vi "Controle_Manip_Main_GUI_Backup2.vi"() -> ()   [LabVIEW 2019] (continued)
                            # "measurement"
                            n1619 = local read "ESP 301 On?"() -> (w2075:bool)
                            n1620 = case shown="True" w2075 {
                              frame False {
                                n1621 = local read "Log file"() -> (w2079:string)
                                n1622 = call "Write2LogFile.vi"("Add to log file"="ESP301 not activated", "Log file before"=w2079, "Checkbox"=FALSE) -> ("Log file after"=w2078:string)
                                n1623 = local write "Log file"(w2078) -> ()
                              }
                              frame True {
                                n1624 = stacked-sequence {
                                frame #0 {
                                # "get refs and exp params"
                                n1625 = local read "LightField Automation out"() -> (w2090:refnum<class "LightField Automation.lvclass">)
                                n1626 = local read "Photodiode error out"() -> (w2085:errorcluster)
                                n1627 = local read "LightField Automation error out"() -> (w2089:errorcluster)
                                n1628 = local read "ESP 301 COM Port"() -> (w2088:refnum<visa-resource-name>)
                                n1629 = local read "Photodiode handle out"() -> (w2086:refnum<visa-resource-name>)
                                n1630 = local read "ESP 301 Error"() -> (w2087:errorcluster)
                                n1631 = property on="Full scale" class="Bool (strict)"("Val(Sgnl)"=TRUE ("Value (Signaling)")) -> ()  [unwired: 2 in, 2 out]
                                n1632 = Bundle("LightField Automation out"=w2090, "LightField Automation error out"=w2089, "ESP 301 COM Port"=w2088, "ESP 301 Error"=w2087, "Photodiode handle out"=w2086, "Photodiode error out"=w2085) -> (→"Test Handles Polar":T16)  [unwired: 1 in]
                                n1633 = local read "CCD ROI"() -> (w2081:T20)
                                n1634 = local read "Exposure Time (ms)"() -> (w2092:dbl)
                                n1635 = local read "Polar Start Angle (°)"() -> (w2096:dbl)
                                n1636 = local read "Polar Step Angle (°)"() -> (w2095:dbl)
                                n1637 = local read "Polar End Angle (°)"() -> (w2091:dbl)
                                n1638 = local read "KCube Shutter On?"() -> (w2084:bool)
                                n1639 = local read "Polar mode"() -> (w2093:u16)
                                n1640 = local read "Acq Mode"() -> (w2094:T3)
                                n1641 = Bundle("Polar End Angle (°)"=w2091, "Polar Start Angle (°)"=w2096, "Polar Step Angle (°)"=w2095, "Acq Mode"=w2094, "Polar mode"=w2093, "Exposure Time (ms)"=w2092, "CCD ROI"=w2081, "KCube Shutter On?"=w2084) -> (→"Polar Params SubVIv2":T15)  [unwired: 1 in]
                                }
                                frame #1 {
                                # "Prepare graph and controls"
                                n1642 = local read "Scan Polarisation References"() -> (w2100:T17)
                                n1643 = local read "Polar Params SubVIv2"() -> (w2101:T15)
                                n1644 = local read "Scan Polar Params"() -> (w2102:refnum<vi>[])
                                n1645 = call "SubVI_PrePolarisation.vi"("Test References"=w2100, "Polar Params SubVIv2"=w2101, "Scan Polar Params"=w2102) -> ()
                                n1646 = property on="Elapsed (s)" class="DigNum (strict)"("Visible"=TRUE) -> ()  [unwired: 2 in, 2 out]
                                n1647 = property on="CCD 1D Spectrum Main" class="XYGraph (strict)"() -> ("XScale.Maximum"=w2105:dbl, "XScale.Minimum"=w2104:dbl, "YScale.Minimum"=w2099:dbl, "YScale.Maximum"=w2103:dbl)  [unwired: 2 in, 2 out]
                                n1648 = property on="Experiment Graph Controls" class="TabCtl (strict)"("Value"=T25."Polar" ("Experiment Graph Controls")) -> ()  [unwired: 2 in, 2 out]
                                n1649 = property on="Polarisation 1D Spectrum" class="XYGraph (strict)"("XScale.Maximum"=w2105, "XScale.Minimum"=w2104, "YScale.Minimum"=w2099, "YScale.Maximum"=w2103) -> ()  [unwired: 2 in, 2 out]
                                }
                                frame #2 {
                                # "actual exp"
                                n1650 = local read "Scan Polarisation References"() -> (w2112:T17)
                                n1651 = local read "Polar Params SubVIv2"() -> (w2113:T15)
                                n1652 = local read "Test Handles Polar"() -> (w2111:T16)
                                n1653 = call "Polarisation_v2.vi"("Test Handles Polar"=w2111, "Polar Params SubVIv2"=w2113, "Test References"=w2112) -> ("2D Pol Data"=w2110:dbl[][], "Test Handles Out"=w2108:T35, "Angles"=w2109:dbl[], "Wavelengths"=w2106:dbl[], "Puissances"=→"PuissancesPolar":dbl[])  [unwired: 1 in]
                                n1654 = local write "Test Handles Polar"(w2108) -> ()
                                n1655 = local write "Angles"(w2109) -> ()
                                n1656 = local write "Wavelength calibration"(w2106) -> ()
                                n1657 = local write "Pol 2D Array Out"(w2110) -> ()
                                }
                                frame #3 {
                                n1658 = control-ref of="MasterStop"() -> (w2115:refnum<vi>)
                                n1659 = control-ref of="MasterPause"() -> (w2116:refnum<vi>)
                                n1660 = control-ref of="ExperimentStopped?"() -> (w2114:refnum<vi>)
                                n1661 = call "CheckStopAndReset.vi"("ExperimentStopped?"=w2114, "MasterStop"=w2115, "MasterPause"=w2116) -> ()
                                }
                                frame #4 {
                                # "end exp"
                                n1662 = local read "Scan Polarisation References"() -> (w2122:T17)
                                n1663 = local read "Scan Polar Params"() -> (w2123:refnum<vi>[])
                                n1664 = local read "Angles"() -> (w2124:dbl[])
                                n1665 = local read "Test Handles Polar"() -> (w2121:T16)
                                n1666 = call "SubVI_PostPolarisation.vi"("Test References"=w2122, "Angles"=w2124, "Scan Polar Params"=w2123) -> ()
                                n1667 = Unbundle By Name(w2121) -> ("LightField Automation out"=w2120:refnum<class "LightField Automation.lvclass">, "LightField Automation error out"=w2119:errorcluster)
                                n1668 = property on="Elapsed (s)" class="DigNum (strict)"("Visible"=FALSE) -> ()  [unwired: 2 in, 2 out]
                                n1669 = local write "LightField Automation error out"(w2119) -> ()
                                n1670 = local write "LightField Automation out"(w2120) -> ()
                                n1671 = property on="Experiment Graph Controls" class="TabCtl (strict)"("Value"=T25."Polar" ("Experiment Graph Controls")) -> ()  [unwired: 2 in, 2 out]
                                }
                                }
                              }
                            }
                          }
                        }
                      }
                      frame "Acquire Contrast" {
                        n1672 = stacked-sequence {
                          frame #0 {
                            # "background"
                            n1673 = local read "Background taken?"() -> (w2125:bool)
                            n1674 = case shown="False" w2125 {
                              frame False {
                                n1675 = stacked-sequence {
                                tunnel: [_ _ w2175] -> w2126
                                frame #0 {
                                n1676 = local read "Log file"() -> (w2160:string)
                                n1677 = property on="CCD 1D Spectrum Main" class="XYGraph (strict)"("YScale.Offset"=0.0 ("Y Scale.Offset and Multiplier:Offset")) -> ()  [unwired: 2 in, 2 out]
                                n1678 = call "Write2LogFile.vi"("Add to log file"="Acquiring background", "Log file before"=w2160, "Checkbox"=FALSE) -> ("Log file after"=w2159:string)
                                n1679 = local write "Log file"(w2159) -> ()
                                }
                                frame #1 {
                                # "make sure shutter is closed"
                                n1680 = local read "KCube Shutter On?"() -> (w2161:bool)
                                n1681 = control-ref of="Shutter Ctrls"() -> (w2165:refnum<vi>)
                                n1682 = property class="Ring (strict)"(reference=w2165) -> ("Value"=w2164:u16)  [unwired: 1 in, 2 out]
                                n1683 = control-ref of="KCube Shutter Device Reference"() -> (w2166:refnum<vi>)
                                n1684 = Equal?(x=w2164, y=u16 0) -> (x = y?=w2162:bool)
                                n1685 = case shown="False" w2162 {
                                tunnel: w2166 -> [w2169 _]
                                tunnel: w2165 -> [w2168 _]
                                tunnel: w2161 -> [w2167 _]
                                frame False {
                                n1686 = call "Shutter.vi"("KCube Shutter Device Reference 2"=w2169, "Shutter Ctrls 2"=w2168, "Shutter on?"=w2167) -> ()
                                }
                                frame True {
                                }
                                }
                                }
                                frame #2 {
                                # "acquire"
                                n1687 = local read "LightField Automation error out"() -> (w2173:errorcluster)
                                n1688 = local read "LightField Automation out"() -> (w2174:refnum<class "LightField Automation.lvclass">)
                                n1689 = local read "Accumulations"() -> (w2170:dbl)
                                n1690 = call "LFA_Capture.vi"("error in (no error)"=w2173, "Frames"=w2170, "LightField Automation in"=w2174) -> ("error out"=w2172:errorcluster, "Data"=w2175:T26, "LightField Automation out"=w2171:refnum<class "LightField Automation.lvclass">)  [unwired: 6 in]
                                n1691 = local write "LightField Automation error out"(w2172) -> ()
                                n1692 = local write "LightField Automation out"(w2171) -> ()
                                }
                                }
                                n1693 = local read "Acq Mode"() -> (w2127:T3)
                                n1694 = case shown="\"Spectrum\", Default" w2127 {
                                selector: w2127 -> [w2128 w2146]
                                tunnel: w2126 -> [w2129 w2147]
                                frame "Spectrum", Default {
                                n1695 = stacked-sequence {
                                tunnel: w2129 -> [_ w2140 _ _]
                                tunnel: w2128 -> [_ w2138 _ _]
                                frame #0 {
                                n1696 = property on="CCD 2D Image Main" class="IntGraph (strict)"("Visible"=FALSE) -> ()  [unwired: 2 in, 2 out]
                                n1697 = property on="CCD 1D Spectrum Main" class="XYGraph (strict)"("Visible"=TRUE) -> ()  [unwired: 2 in, 2 out]
                                }
                                frame #1 {
                                n1698 = local read "Wavelength calibration"() -> (w2137:dbl[])
                                n1699 = local read "CCD ROI"() -> (w2133:T20)
                                n1700 = Divide(x=1239.842, y=w2137) -> (x/y=w2135:dbl[])
                                n1701 = call "PrepareData4Graph.vi"("Wavelength nm"=w2135, "DataLF"=w2140, "CCD ROI"=w2133, "AcqMode"=w2138, "Data type"=T30."Spectre") -> ("Spectrum"=w2139:cluster{"Array 2":dbl[], "Array":dbl[]}, "PLInt out"=w2132:dbl[])  [unwired: 2 in, 2 out]
                                n1702 = local write "CCD 1D Spectrum Main"(w2139) -> ()
                                n1703 = local write "BackgroundSpec"(w2132) -> ()
                                }
                                frame #2 {
                                n1704 = local read "BackgroundSpec"() -> (w2141:dbl[])
                                n1705 = call-poly <vilib>:"Mean.vi"("X"=w2141) -> ("mean"=w2143:dbl)  [unwired: 1 out]
                                n1706 = Negate(x=w2143) -> (-x=w2142:dbl)
                                n1707 = property on="CCD 1D Spectrum Main" class="XYGraph (strict)"("YScale.Offset"=w2142) -> ()  [unwired: 2 in, 2 out]
                                }
                                frame #3 {
                                n1708 = local write "Background taken?"(TRUE ("Background taken?")) -> ()
                                n1709 = property on="Background substract" class="Enum (strict)"("Value"=enum16{"None", "Shutter"}."None" ("Background substract")) -> ()  [unwired: 2 in, 2 out]
                                }
                                }
                                }
                                frame "Image" {
                                n1710 = stacked-sequence {
                                tunnel: w2147 -> [_ w2155]
                                tunnel: w2146 -> [_ w2153]
                                frame #0 {
                                n1711 = property on="CCD 1D Spectrum Main" class="XYGraph (strict)"("Visible"=FALSE) -> ()  [unwired: 2 in, 2 out]
                                n1712 = property on="CCD 2D Image Main" class="IntGraph (strict)"("Visible"=TRUE) -> ()  [unwired: 2 in, 2 out]
                                }
                                frame #1 {
                                n1713 = local read "Wavelength calibration"() -> (w2154:dbl[])
                                n1714 = local read "CCD ROI"() -> (w2150:T20)
                                n1715 = call "PrepareData4Graph.vi"("Wavelength nm"=w2154, "DataLF"=w2155, "CCD ROI"=w2150, "AcqMode"=w2153, "Data type"=T30."Spectre") -> ("Intensity Graph"=w2152:dbl[][])  [unwired: 2 in, 3 out]
                                n1716 = local write "CCD 2D Image Main"(w2152) -> ()
                                }
                                }
                                }
                                }
                              }
                              frame True {
                              }
                            }
                          }
                          frame #1 {
                            # "measurement"
                            n1717 = stacked-sequence {
                              frame #0 {
                                w2178 = FALSE ("Value")
                                w2179 = TRUE ("Visible")
                                w2183 = FALSE
                                w2188 = FALSE ("Acq Cont")
                                n1718 = property on="CCD 1D Spectrum Main" class="XYGraph (strict)"() -> ("XScale.Maximum"=w2187:dbl, "XScale.Minimum"=w2186:dbl, "YScale.Minimum"=w2185:dbl, "YScale.Maximum"=w2184:dbl)  [unwired: 2 in, 2 out]
                                n1719 = property on="Acquire Contrast" class="Bool (strict)"("Visible"=w2183) -> ()  [unwired: 2 in, 2 out]
                                n1720 = property on="Save Contrast" class="Bool (strict)"("Visible"=w2183) -> ()  [unwired: 2 in, 2 out]
                                n1721 = property on="Contrast 1D Spectrum" class="XYGraph (strict)"("XScale.Maximum"=w2187, "XScale.Minimum"=w2186, "YScale.Minimum"=w2185, "YScale.Maximum"=w2184) -> ()  [unwired: 2 in, 2 out]
                                n1722 = local read "Scan Contrast Ctrls"() -> (w2191:refnum<vi>[])
                                n1723 = property on="Scan Linear Stage Progess Bar" class="Slide (strict)"("Visible"=TRUE, "Value"=u8 0 ("Scan Linear Stage Progess Bar")) -> ()  [unwired: 2 in, 2 out]
                                n1724 = local write "Acquire Contrast"(w2188) -> ()
                                n1725 = local write "Save Contrast"(w2188) -> ()
                                n1726 = call "Enable&Disable_Controls.vi"("Enum"=enum16{"Enabled", "Disabled", "Disabled&Grayed"}."Disabled&Grayed", "References"=w2191) -> ()  [unwired: 1 in]
                                n1727 = property on="Scan Linear Stage Progess Bar" class="Slide (strict)"("Visible"=TRUE) -> ()  [unwired: 2 in, 2 out]
                                n1728 = property on="Elapsed (s)" class="DigNum (strict)"("Visible"=TRUE) -> ()  [unwired: 2 in, 2 out]
                                n1729 = control-ref of="MasterStop"() -> (w2181:refnum<vi>)
                                n1730 = control-ref of="MasterPause"() -> (w2180:refnum<vi>)
                                n1731 = property on="Experiment Graph Controls" class="TabCtl (strict)"("Value"=T25."Contrast" ("Experiment Graph Controls")) -> ()  [unwired: 2 in, 2 out]
                                n1732 = property class="Bool (strict)"(reference=w2180, "Visible"=w2179, "Value"=w2178) -> ()  [unwired: 1 in, 2 out]
                                n1733 = property class="Bool (strict)"(reference=w2181, "Visible"=w2179, "Value"=w2178) -> ()  [unwired: 1 in, 2 out]
                              }
                              frame #1 {
                                n1734 = local read "Excitation Wavelength (nm)"() -> (w2197:dbl)
                                n1735 = local read "LinTFines Step Pos (usteps)"() -> (w2202:dbl)
                                n1736 = local read "LinTFine Start Pos (usteps)"() -> (w2203:dbl)
                                n1737 = local read "LinTFine End Pos (usteps)"() -> (w2201:dbl)
                                n1738 = local read "Exposure Time (ms)"() -> (w2199:dbl)
                                n1739 = local read "LinT Start Pos (mm)"() -> (w2206:dbl)
                                n1740 = local read "LinT Step Pos (mm)"() -> (w2205:dbl)
                                n1741 = local read "LinT End pos (mm)"() -> (w2204:dbl)
                                n1742 = local read "KCube Shutter On?"() -> (w2194:bool)
                                n1743 = local read "Accumulations"() -> (w2198:dbl)
                                n1744 = local read "Acq Mode"() -> (w2196:T3)
                                n1745 = local read "CCD ROI"() -> (w2195:T20)
                                n1746 = Bundle("LinT Start Pos (mm)"=w2206, "LinT Step Pos (mm)"=w2205, "LinT End pos (mm)"=w2204, "LinTFine Start Pos (usteps)"=w2203, "LinTFines Step Pos (usteps)"=w2202, "LinTFine End Pos (usteps)"=w2201) -> (w2200:T27)  [unwired: 1 in]
                                n1747 = Bundle("Exposure Time (ms)"=w2199, "Accumulations"=w2198, "Excitation Wavelength (nm)"=w2197, "Acq Mode"=w2196, "CCD ROI"=w2195, "KCube Shutter On?"=w2194) -> (w2193:T24)  [unwired: 1 in]
                                n1748 = local write "Scan Translation Params"(w2200) -> ()
                                n1749 = local write "Scan Translation Exp Params"(w2193) -> ()
                              }
                              frame #2 {
                                n1750 = local read "Scan Translation Exp Params"() -> (w2214:T24)
                                n1751 = local read "Scan Translation Params"() -> (w2231:T27)
                                n1752 = control-ref of="Scan Linear Stage Progess Bar"() -> ()  [unwired: 1 out]
                                n1753 = control-ref of="Stop Contrast"() -> ()  [unwired: 1 out]
                                n1754 = local read "ESP 301 COM Port"() -> (w2224:refnum<visa-resource-name>)
                                n1755 = control-ref of="Pause Contrast"() -> ()  [unwired: 1 out]
                                n1756 = control-ref of="Scan Main Progess Bar"() -> (w2213:refnum<vi>)
                                n1757 = local read "LightField Automation error out"() -> (w2211:errorcluster)
                                n1758 = local read "ESP 301 Error"() -> (w2226:errorcluster)
                                n1759 = local read "LightField Automation out"() -> (w2212:refnum<class "LightField Automation.lvclass">)
                                n1760 = control-ref of="Shutter Ctrls"() -> (w2216:refnum<vi>)
                                n1761 = control-ref of="KCube Shutter Device Reference"() -> (w2217:refnum<vi>)
                                n1762 = control-ref of="PZC Position Readout (usteps)"() -> (w2215:refnum<vi>)
                                n1763 = control-ref of="Contrast 1D Spectrum"() -> (w2218:refnum<vi>)
                                n1764 = control-ref of="Contrast Oscillations"() -> (w2219:refnum<vi>)
                                n1765 = Open VI Reference(type specifier VI Refnum (for type only)=refnum<vi> refnum ("application reference (local)"), vi path=path "C:/Users/manip/Documents/Controle_Manip_2020/subVIs/Scans/FineContrast_cleaned inputs.vi", options=256) -> (vi reference=w2229:refnum<vi>, error out=w2238:errorcluster)  [unwired: 3 in]
                                n1766 = local read "PZC200 Instrument Channel"() -> (w2230:string)
                                n1767 = call-by-ref "Wait On Asynchronous Call"(reference=w2229, error in=w2238) -> (reference out=w2237:refnum<vi>, error out=w2236:errorcluster, "PZAPos & InstPow"=w2227:dbl[][], "Spectra vs PZA"=w2234:i32[][], "LFA out"=w2210:refnum<class "LightField Automation.lvclass">, "PZC out"=w2228:string, "Photodiode out"=w2220:refnum<visa-resource-name>, "ESP 301 COM out"=w2223:refnum<visa-resource-name>, "LFA error out"=w2209:errorcluster, "PZC error out"=w2221:errorcluster, "Photodiode error out"=w2222:errorcluster, "ESP 301 error out"=w2225:errorcluster)  [unwired: 18 in]
                                n1768 = local write "PZAPos&Pow"(w2227) -> ()
                                n1769 = local write "Photodiode error out"(w2222) -> ()
                                n1770 = local write "PZC200 Instrument Channel"(w2228) -> ()
                                n1771 = local write "Contrast Array Out"(w2234) -> ()
                                n1772 = local read "PZC Error"() -> (w2235:errorcluster)
                                n1773 = local write "ESP 301 COM Port"(w2223) -> ()
                                n1774 = Close Reference(reference=w2237, error in (no error)=w2236) -> ()  [unwired: 1 out]
                                n1775 = local write "Photodiode handle out"(w2220) -> ()
                                n1776 = local read "Photodiode handle out"() -> (w2232:refnum<visa-resource-name>)
                                n1777 = local write "ESP 301 Error"(w2225) -> ()
                                n1778 = local read "Photodiode error out"() -> (w2233:errorcluster)
                                n1779 = local write "LightField Automation error out"(w2209) -> ()
                                n1780 = local write "LightField Automation out"(w2210) -> ()
                                n1781 = local write "PZC Error"(w2221) -> ()
                                n1782 = control-ref of="MasterStop"() -> (w2207:refnum<vi>)
                                n1783 = control-ref of="MasterPause"() -> (w2208:refnum<vi>)
                                n1784 = call-by-ref "Start Asynchronous Call"(reference=w2229, error in=w2238, "LFA in"=w2212, "PZC in"=w2230, "Photodiode in"=w2232, "ESP 301 COM"=w2224, "LFA error in"=w2211, "PZC error in"=w2235, "Photodiode error in"=w2233, "ESP 301 error in"=w2226, "Scan Translation Exp Params"=w2214, "PZC Pos (usteps)"=w2215, "Scan Translation Params"=w2231, "Pause button"=w2208, "Contrast Oscillations"=w2219, "Stop button"=w2207, "Contrast 1D Spectrum"=w2218, "Progess Bar"=w2213, "Shutter Device"=w2217, "Shutter"=w2216) -> ()  [unwired: 12 out]
                              }
                              frame #3 {
                                w2254 = FALSE ("Acq Cont")
                                w2251 = FALSE ("Acq Cont")
                                n1785 = local read "Auto< ?"() -> (w2249:bool)
                                n1786 = property on="Scan Linear Stage Progess Bar" class="Slide (strict)"("Visible"=FALSE, "Value"=u8 0 ("Scan Linear Stage Progess Bar")) -> ()  [unwired: 2 in, 2 out]
                                n1787 = Not(x=w2249) -> (.not. x?=w2248:bool)
                                n1788 = local write "Pause Michelson"(w2254) -> ()
                                n1789 = local write "Stop Michelson"(w2254) -> ()
                                n1790 = property on="Save Contrast" class="Bool (strict)"("Visible"=w2248) -> ()  [unwired: 2 in, 2 out]
                                n1791 = property on="Acquire Contrast" class="Bool (strict)"("Visible"=TRUE) -> ()  [unwired: 2 in, 2 out]
                                n1792 = local write "Acquire Michelson"(w2251) -> ()
                                n1793 = local write "Acquire Contrast"(w2251) -> ()
                                n1794 = local write "Save Michelson"(w2251) -> ()
                                n1795 = local read "Scan Contrast Ctrls"() -> (w2247:refnum<vi>[])
                                n1796 = property on="Elapsed (s)" class="DigNum (strict)"("Visible"=FALSE) -> ()  [unwired: 2 in, 2 out]
                                n1797 = control-ref of="MasterStop"() -> (w2244:refnum<vi>)
                                n1798 = control-ref of="MasterPause"() -> (w2245:refnum<vi>)
                                n1799 = call "Enable&Disable_Controls.vi"("Enum"=enum16{"Enabled", "Disabled", "Disabled&Grayed"}."Enabled", "References"=w2247) -> ()  [unwired: 1 in]
                                n1800 = control-ref of="ExperimentStopped?"() -> (w2243:refnum<vi>)
                                n1801 = call "CheckStopAndReset.vi"("ExperimentStopped?"=w2243, "MasterStop"=w2244, "MasterPause"=w2245) -> ()
                              }
                            }
                          }
                        }
                      }
                      frame "Acquire Michelson" {
                        n1802 = stacked-sequence {
                          frame #0 {
                            # "background"
                            n1803 = local read "Background taken?"() -> (w2255:bool)
                            n1804 = case shown="False" w2255 {
                              frame False {
                                n1805 = stacked-sequence {
                                tunnel: [_ _ w2305] -> w2256
                                frame #0 {
                                n1806 = local read "Log file"() -> (w2290:string)
                                n1807 = property on="CCD 1D Spectrum Main" class="XYGraph (strict)"("YScale.Offset"=0.0 ("Y Scale.Offset and Multiplier:Offset")) -> ()  [unwired: 2 in, 2 out]
                                n1808 = call "Write2LogFile.vi"("Add to log file"="Acquiring background", "Log file before"=w2290, "Checkbox"=FALSE) -> ("Log file after"=w2289:string)
                                n1809 = local write "Log file"(w2289) -> ()
                                }
                                frame #1 {
                                # "make sure shutter is closed"
                                n1810 = local read "KCube Shutter On?"() -> (w2291:bool)
                                n1811 = control-ref of="Shutter Ctrls"() -> (w2295:refnum<vi>)
                                n1812 = property class="Ring (strict)"(reference=w2295) -> ("Value"=w2294:u16)  [unwired: 1 in, 2 out]
                                n1813 = control-ref of="KCube Shutter Device Reference"() -> (w2296:refnum<vi>)
                                n1814 = Equal?(x=w2294, y=u16 0) -> (x = y?=w2292:bool)
                                n1815 = case shown="False" w2292 {
                                tunnel: w2296 -> [w2299 _]
                                tunnel: w2295 -> [w2298 _]
                                tunnel: w2291 -> [w2297 _]
                                frame False {
                                n1816 = call "Shutter.vi"("KCube Shutter Device Reference 2"=w2299, "Shutter Ctrls 2"=w2298, "Shutter on?"=w2297) -> ()
                                }
                                frame True {
                                }
                                }
                                }
                                frame #2 {
                                # "acquire"
                                n1817 = local read "LightField Automation error out"() -> (w2303:errorcluster)
                                n1818 = local read "LightField Automation out"() -> (w2304:refnum<class "LightField Automation.lvclass">)
                                n1819 = local read "Accumulations"() -> (w2300:dbl)
                                n1820 = call "LFA_Capture.vi"("error in (no error)"=w2303, "Frames"=w2300, "LightField Automation in"=w2304) -> ("error out"=w2302:errorcluster, "Data"=w2305:T26, "LightField Automation out"=w2301:refnum<class "LightField Automation.lvclass">)  [unwired: 6 in]
                                n1821 = local write "LightField Automation error out"(w2302) -> ()
                                n1822 = local write "LightField Automation out"(w2301) -> ()
                                }
                                }
                                n1823 = local read "Acq Mode"() -> (w2257:T3)
                                n1824 = case shown="\"Spectrum\", Default" w2257 {
                                selector: w2257 -> [w2258 w2276]
                                tunnel: w2256 -> [w2259 w2277]
                                frame "Spectrum", Default {
                                n1825 = stacked-sequence {
                                tunnel: w2259 -> [_ w2270 _ _]
                                tunnel: w2258 -> [_ w2268 _ _]
                                frame #0 {
                                n1826 = property on="CCD 2D Image Main" class="IntGraph (strict)"("Visible"=FALSE) -> ()  [unwired: 2 in, 2 out]
                                n1827 = property on="CCD 1D Spectrum Main" class="XYGraph (strict)"("Visible"=TRUE) -> ()  [unwired: 2 in, 2 out]
                                }
                                frame #1 {
                                n1828 = local read "Wavelength calibration"() -> (w2267:dbl[])
                                n1829 = local read "CCD ROI"() -> (w2263:T20)
                                n1830 = Divide(x=1239.842, y=w2267) -> (x/y=w2265:dbl[])
                                n1831 = call "PrepareData4Graph.vi"("Wavelength nm"=w2265, "DataLF"=w2270, "CCD ROI"=w2263, "AcqMode"=w2268, "Data type"=T30."Spectre") -> ("Spectrum"=w2269:cluster{"Array 2":dbl[], "Array":dbl[]}, "PLInt out"=w2262:dbl[])  [unwired: 2 in, 2 out]
                                n1832 = local write "CCD 1D Spectrum Main"(w2269) -> ()
                                n1833 = local write "BackgroundSpec"(w2262) -> ()
                                }
                                frame #2 {
                                n1834 = local read "BackgroundSpec"() -> (w2271:dbl[])
                                n1835 = call-poly <vilib>:"Mean.vi"("X"=w2271) -> ("mean"=w2273:dbl)  [unwired: 1 out]
                                n1836 = Negate(x=w2273) -> (-x=w2272:dbl)
                                n1837 = property on="CCD 1D Spectrum Main" class="XYGraph (strict)"("YScale.Offset"=w2272) -> ()  [unwired: 2 in, 2 out]
                                }
                                frame #3 {
                                n1838 = local write "Background taken?"(TRUE ("Background taken?")) -> ()
                                n1839 = property on="Background substract" class="Enum (strict)"("Value"=enum16{"None", "Shutter"}."None" ("Background substract")) -> ()  [unwired: 2 in, 2 out]
                                }
                                }
                                }
                                frame "Image" {
                                n1840 = stacked-sequence {
                                tunnel: w2277 -> [_ w2285]
                                tunnel: w2276 -> [_ w2283]
                                frame #0 {
                                n1841 = property on="CCD 1D Spectrum Main" class="XYGraph (strict)"("Visible"=FALSE) -> ()  [unwired: 2 in, 2 out]
                                n1842 = property on="CCD 2D Image Main" class="IntGraph (strict)"("Visible"=TRUE) -> ()  [unwired: 2 in, 2 out]
                                }
                                frame #1 {
                                n1843 = local read "Wavelength calibration"() -> (w2284:dbl[])
                                n1844 = local read "CCD ROI"() -> (w2280:T20)
                                n1845 = call "PrepareData4Graph.vi"("Wavelength nm"=w2284, "DataLF"=w2285, "CCD ROI"=w2280, "AcqMode"=w2283, "Data type"=T30."Spectre") -> ("Intensity Graph"=w2282:dbl[][])  [unwired: 2 in, 3 out]
                                n1846 = local write "CCD 2D Image Main"(w2282) -> ()
                                }
                                }
                                }
                                }
                              }
                              frame True {
                              }
                            }
                          }
                          frame #1 {
                            # "measurement"
                            n1847 = Get Date/Time In Seconds() -> (seconds since 1Jan1904=w2306:timestamp)
                            n1848 = stacked-sequence {
                              tunnel: w2306 -> [_ _ w2340 w2464]
                              frame #0 {
                                w2312 = TRUE
                                w2313 = FALSE ("Acq Cont")
                                w2310 = TRUE
                                w2309 = FALSE
                                w2311 = FALSE
                                # "check that range is within translation stage travel"
                                # "get params and check feasability"
                                n1849 = property on="Save Michelson" class="Bool (strict)"("Visible"=w2311) -> ()  [unwired: 2 in, 2 out]
                                n1850 = property on="Pause Michelson" class="Bool (strict)"("Visible"=w2310) -> ()  [unwired: 2 in, 2 out]
                                n1851 = property on="Save Contrast" class="Bool (strict)"("Visible"=w2311) -> ()  [unwired: 2 in, 2 out]
                                n1852 = property on="Pause Contrast" class="Bool (strict)"("Visible"=w2310) -> ()  [unwired: 2 in, 2 out]
                                n1853 = property on="Stop Contrast" class="Bool (strict)"("Visible"=w2310) -> ()  [unwired: 2 in, 2 out]
                                n1854 = property on="Acquire Michelson" class="Bool (strict)"("Visible"=w2311) -> ()  [unwired: 2 in, 2 out]
                                n1855 = property on="Stop Michelson" class="Bool (strict)"("Visible"=w2310) -> ()  [unwired: 2 in, 2 out]
                                n1856 = property on="Acquire Contrast" class="Bool (strict)"("Visible"=w2311) -> ()  [unwired: 2 in, 2 out]
                                n1857 = property on="Scan Linear Stage Progess Bar" class="Slide (strict)"("Visible"=TRUE, "Value"=u8 0 ("Scan Linear Stage Progess Bar")) -> ()  [unwired: 2 in, 2 out]
                                n1858 = property on="Scan Michelson Progess Bar" class="Slide (strict)"("Value"=u8 0 ("Scan Michelson Progess Bar"), "Visible"=TRUE) -> ()  [unwired: 2 in, 2 out]
                                n1859 = local read "Scan Contrast Ctrls"() -> (w2319:refnum<vi>[])
                                n1860 = local write "Acquire Contrast"(w2313) -> ()
                                n1861 = local write "Save Contrast"(w2313) -> ()
                                n1862 = call "Enable&Disable_Controls.vi"("Enum"=enum16{"Enabled", "Disabled", "Disabled&Grayed"}."Disabled&Grayed", "References"=w2319) -> ()  [unwired: 1 in]
                                n1863 = property on="Michelson Expected (s)" class="DigNum (strict)"("Visible"=w2312) -> ()  [unwired: 2 in, 2 out]
                                n1864 = property on="Elapsed (s)" class="DigNum (strict)"("Visible"=TRUE) -> ()  [unwired: 2 in, 2 out]
                                n1865 = property on="Experiment Graph Controls" class="TabCtl (strict)"("Value"=T25."Contrast" ("Experiment Graph Controls")) -> ()  [unwired: 2 in, 2 out]
                                n1866 = property on="Michelson Elapsed (s)" class="DigNum (strict)"("Visible"=w2312) -> ()  [unwired: 2 in, 2 out]
                                n1867 = local write "Acquire Michelson"(w2309) -> ()
                                n1868 = local write "Save Michelson"(w2309) -> ()
                              }
                              frame #1 {
                                # "check that range is within translation stage travel"
                                # "get params"
                                n1869 = local read "Excitation Wavelength (nm)"() -> (w2324:dbl)
                                n1870 = local read "Exposure Time (ms)"() -> (w2326:dbl)
                                n1871 = local read "KCube Shutter On?"() -> (w2321:bool)
                                n1872 = local read "Accumulations"() -> (w2325:dbl)
                                n1873 = local read "Acq Mode"() -> (w2323:T3)
                                n1874 = local read "CCD ROI"() -> (w2322:T20)
                                n1875 = local read "LinTFines Step Pos (usteps)"() -> (w2329:dbl)
                                n1876 = local read "LinTFine Start Pos (usteps)"() -> (w2330:dbl)
                                n1877 = local read "LinTFine End Pos (usteps)"() -> (w2328:dbl)
                                n1878 = local read "LinT Start Pos (mm)"() -> (w2333:dbl)
                                n1879 = local read "LinT Step Pos (mm)"() -> (w2332:dbl)
                                n1880 = local read "LinT End pos (mm)"() -> (w2331:dbl)
                                n1881 = Bundle("Exposure Time (ms)"=w2326, "Accumulations"=w2325, "Excitation Wavelength (nm)"=w2324, "Acq Mode"=w2323, "CCD ROI"=w2322, "KCube Shutter On?"=w2321) -> (w2320:T24)  [unwired: 1 in]
                                n1882 = Bundle("LinT Start Pos (mm)"=w2333, "LinT Step Pos (mm)"=w2332, "LinT End pos (mm)"=w2331, "LinTFine Start Pos (usteps)"=w2330, "LinTFines Step Pos (usteps)"=w2329, "LinTFine End Pos (usteps)"=w2328) -> (w2327:T27)  [unwired: 1 in]
                                n1883 = local write "Scan Translation Exp Params"(w2320) -> ()
                                n1884 = local write "Scan Translation Params"(w2327) -> ()
                              }
                              frame #2 {
                                # "pzc & inst pow"
                                # "esp pos"
                                # "data"
                                # "move ESP"
                                n1885 = local read "LightField Automation out"() -> (w2337:refnum<class "LightField Automation.lvclass">)
                                n1886 = local read "ESP 301 COM Port"() -> (w2339:refnum<visa-resource-name>)
                                n1887 = local read "LinT Start Pos (mm)"() -> (w2350:dbl)
                                n1888 = local read "ESP 301 Error"() -> (w2346:errorcluster)
                                n1889 = local read "LinT Step Pos (mm)"() -> (w2351:dbl)
                                n1890 = local read "LinT End pos (mm)"() -> (w2355:dbl)
                                n1891 = local read "LinT Start Pos (mm)"() -> (w2356:dbl)
                                n1892 = local read "LinT Step Pos (mm)"() -> (w2353:dbl)
                                n1893 = local read "LightField Automation error out"() -> (w2336:errorcluster)
                                n1894 = Subtract(x=w2355, y=w2356) -> (x-y=w2354:dbl)
                                n1895 = Divide(x=w2354, y=w2353) -> (x/y=w2352:dbl)
                                n1896 = Increment(x=w2352) -> (x+1=w2349:dbl)
                                n1897 = for {
                                N: w2349 -> [w2362]
                                tunnel: w2351 -> [w2379]
                                tunnel: w2350 -> [w2378]
                                shift-right: [w2374] -> w2347
                                shift-left: dbl[] [] -> [w2375]
                                shift-right: [w2372] -> w2335
                                shift-left: w2337 -> [w2373]
                                shift-right: [w2370] -> w2334
                                shift-left: w2336 -> [w2371]
                                shift-right: [w2368] -> w2345
                                shift-left: w2346 -> [w2369]
                                shift-right: [w2366] -> w2343
                                shift-left: dbl[][][] [] -> [w2367]
                                shift-right: [w2364] -> w2341
                                shift-left: dbl[][][] [] -> [w2365]
                                tunnel: w2340 -> [w2360]
                                shift-right: [w2357] -> w2338
                                shift-left: w2339 -> [w2358]
                                i -> [w2361]
                                stop <- w2359 stop-if-true
                                # "ESP"
                                n1898 = Multiply(x=w2361, y=w2379) -> (x*y=w2377:dbl)
                                n1899 = Add(x=w2378, y=w2377) -> (x+y=w2376:dbl)
                                n1900 = Divide(x=w2361, y=w2362) -> (x/y=w2363:dbl)
                                n1901 = stacked-sequence {
                                tunnel: w2376 -> [w2384 w2390 _ _]
                                tunnel: w2375 -> [w2386 _ _ _]
                                tunnel: [w2385 _ _ _] -> w2374
                                tunnel: w2373 -> [_ _ w2433 _]
                                tunnel: [_ _ w2432 _] -> w2372
                                tunnel: w2371 -> [_ _ w2431 _]
                                tunnel: [_ _ w2430 _] -> w2370
                                tunnel: w2369 -> [w2383 _ _ _]
                                tunnel: [w2382 _ _ _] -> w2368
                                tunnel: w2367 -> [_ _ w2402 _]
                                tunnel: [_ _ w2400 _] -> w2366
                                tunnel: w2365 -> [_ _ w2399 _]
                                tunnel: [_ _ w2397 _] -> w2364
                                tunnel: w2363 -> [_ _ _ w2443]
                                tunnel: w2362 -> [_ _ _ w2442]
                                tunnel: w2361 -> [_ _ _ w2440]
                                tunnel: w2360 -> [_ _ _ w2441]
                                tunnel: [_ _ _ w2438] -> w2359
                                tunnel: w2358 -> [w2381 _ _ _]
                                tunnel: [w2380 _ _ _] -> w2357
                                frame #0 {
                                # "pos readout"
                                n1902 = control-ref of="Newport Linear Translation Stage Position Readout (mm)"() -> (w2387:refnum<vi>)
                                n1903 = call "ESP301_Go2Pos.vi"("VISA resource name"=w2381, "Set value"=w2384, "Axis (1)"=1, "Error In"=w2383, "DigNum Refnum"=w2387) -> ("VISA resource name 2"=w2380:refnum<visa-resource-name>, "Error In 2"=w2382:errorcluster)
                                n1904 = Insert Into Array(array=w2386, new element=w2384) -> (w2385:dbl[])  [unwired: 1 in]
                                }
                                frame #1 {
                                # "wait on ESP"
                                n1905 = Wait (ms)(milliseconds to wait=u32 50) -> ()  [unwired: 1 out]
                                n1906 = Number To Decimal String(number=w2390) -> (decimal integer string=w2393:string)  [unwired: 1 in]
                                n1907 = local read "Log file"() -> (w2396:string)
                                n1908 = Concatenate Strings("ESP moved to ", w2393) -> (w2392:string)
                                n1909 = call "Write2LogFile.vi"("Add to log file"=w2392, "Log file before"=w2396, "Checkbox"=FALSE) -> ("Log file after"=w2395:string)
                                n1910 = local write "Log file"(w2395) -> ()
                                }
                                frame #2 {
                                n1911 = control-ref of="Shutter Ctrls"() -> (w2420:refnum<vi>)
                                n1912 = control-ref of="Scan Linear Stage Progess Bar"() -> (w2416:refnum<vi>)
                                n1913 = control-ref of="KCube Shutter Device Reference"() -> (w2421:refnum<vi>)
                                n1914 = control-ref of="PZC Position Readout (usteps)"() -> (w2419:refnum<vi>)
                                n1915 = control-ref of="Pause Contrast"() -> (w2418:refnum<vi>)
                                n1916 = control-ref of="Contrast 1D Spectrum"() -> (w2422:refnum<vi>)
                                n1917 = control-ref of="Contrast Oscillations"() -> (w2423:refnum<vi>)
                                n1918 = local read "Photodiode handle out"() -> (w2412:refnum<visa-resource-name>)
                                n1919 = local read "Photodiode error out"() -> (w2413:errorcluster)
                                n1920 = control-ref of="Stop Contrast"() -> (w2417:refnum<vi>)
                                n1921 = local read "Scan Translation Params"() -> (w2425:T27)
                                n1922 = Open VI Reference(type specifier VI Refnum (for type only)=refnum<vi> refnum ("application reference (local)"), vi path=path "C:/Users/manip/Documents/Controle_Manip_2020/subVIs/Scans/FineContrast_cleaned inputs.vi", options=256) -> (vi reference=w2427:refnum<vi>, error out=w2426:errorcluster)  [unwired: 3 in]
                                n1923 = local read "Scan Translation Exp Params"() -> (w2424:T24)
                                n1924 = local read "PZC200 Instrument Channel"() -> (w2411:string)
                                n1925 = local read "ESP 301 Error"() -> (w2414:errorcluster)
                                n1926 = local read "PZC Error"() -> (w2410:errorcluster)
                                n1927 = local read "ESP 301 COM Port"() -> (w2415:refnum<visa-resource-name>)
                                n1928 = call-by-ref "Start Asynchronous Call"(reference=w2427, error in=w2426, "LFA in"=w2433, "PZC in"=w2411, "Photodiode in"=w2412, "ESP 301 COM"=w2415, "LFA error in"=w2431, "PZC error in"=w2410, "Photodiode error in"=w2413, "ESP 301 error in"=w2414, "Scan Translation Exp Params"=w2424, "PZC Pos (usteps)"=w2419, "Scan Translation Params"=w2425, "Pause button"=w2418, "Contrast Oscillations"=w2423, "Stop button"=w2417, "Contrast 1D Spectrum"=w2422, "Progess Bar"=w2416, "Shutter Device"=w2421, "Shutter"=w2420) -> ()  [unwired: 12 out]
                                n1929 = call-by-ref "Wait On Asynchronous Call"(reference=w2427, error in=w2426) -> ("PZAPos & InstPow"=w2398:dbl[][], "Spectra vs PZA"=w2401:i32[][], "LFA out"=w2432:refnum<class "LightField Automation.lvclass">, "PZC out"=w2407:string, "Photodiode out"=w2406:refnum<visa-resource-name>, "ESP 301 COM out"=w2408:refnum<visa-resource-name>, "LFA error out"=w2430:errorcluster, "PZC error out"=w2404:errorcluster, "Photodiode error out"=w2405:errorcluster, "ESP 301 error out"=w2409:errorcluster)  [unwired: 18 in, 2 out]
                                n1930 = local write "PZC200 Instrument Channel"(w2407) -> ()
                                n1931 = local write "Photodiode handle out"(w2406) -> ()
                                n1932 = local write "Photodiode error out"(w2405) -> ()
                                n1933 = local write "ESP 301 COM Port"(w2408) -> ()
                                n1934 = Insert Into Array(array=w2399, new element=w2398) -> (w2397:dbl[][][])  [unwired: 3 in]
                                n1935 = local write "ESP 301 Error"(w2409) -> ()
                                n1936 = local write "PZC Error"(w2404) -> ()
                                n1937 = Insert Into Array(array=w2402, new element=w2401) -> (w2400:dbl[][][])  [unwired: 3 in]
                                }
                                frame #3 {
                                n1938 = local read "Pause Michelson"() -> (w2437:bool)
                                n1939 = control-ref of="Expected (s)"() -> (w2435:refnum<vi>)
                                n1940 = Increment(x=w2440) -> (x+1=w2439:i32)
                                n1941 = Multiply(x=w2443, y=100.0) -> (x*y=w2445:dbl)
                                n1942 = call "Expectedtime.vi"("N"=w2442, "I"=w2439, "Reference time"=w2441) -> ("Expected time"=w2434:dbl, "Elapsed time"=w2436:dbl)
                                "Michelson Elapsed (s)" <- w2436
                                "Michelson Expected (s)" <- w2434
                                n1943 = property class="DigNum (strict)"(reference=w2435, "Value"=w2434) -> ()  [unwired: 1 in, 2 out]
                                n1944 = property on="Elapsed (s)" class="DigNum (strict)"("Value"=w2436) -> ()  [unwired: 2 in, 2 out]
                                n1945 = local write "Scan Michelson Progess Bar"(w2445) -> ()
                                n1946 = case shown="True" w2437 {
                                frame False {
                                }
                                frame True {
                                n1947 = while {
                                stop <- w2447 stop-if-true
                                n1948 = local read "Pause Michelson"() -> (w2448:bool)
                                n1949 = Wait (ms)(milliseconds to wait=u32 50) -> ()  [unwired: 1 out]
                                n1950 = Not(x=w2448) -> (.not. x?=w2447:bool)
                                }
                                }
                                }
                                n1951 = local read "Stop Michelson"() -> (w2438:bool)
                                }
                                }
                                }
                                "ESP Pos" <- w2347
                                "PZC&Pow3D" <- w2341
                                n1952 = local write "LightField Automation error out"(w2334) -> ()
                                n1953 = local write "LightField Automation out"(w2335) -> ()
                                n1954 = local write "ESP 301 COM Port"(w2338) -> ()
                                n1955 = local write "Michelson Array Out"(w2343) -> ()
                                n1956 = local write "ESP 301 Error"(w2345) -> ()
                              }
                              frame #3 {
                                w2456 = FALSE
                                w2458 = FALSE
                                w2455 = FALSE ("Visible")
                                n1957 = Get Date/Time In Seconds() -> (seconds since 1Jan1904=w2465:timestamp)
                                n1958 = property on="Scan Linear Stage Progess Bar" class="Slide (strict)"("Visible"=FALSE) -> ()  [unwired: 2 in, 2 out]
                                n1959 = Subtract(x=w2465, y=w2464) -> (x-y=w2463:dbl)
                                n1960 = property on="Stop Michelson" class="Bool (strict)"("Visible"=w2456) -> ()  [unwired: 2 in, 2 out]
                                n1961 = property on="Pause Michelson" class="Bool (strict)"("Visible"=w2456) -> ()  [unwired: 2 in, 2 out]
                                n1962 = local write "Michelson Elapsed (s)"(w2463) -> ()
                                n1963 = local read "Auto< ?"() -> (w2454:bool)
                                n1964 = Not(x=w2454) -> (.not. x?=w2453:bool)
                                n1965 = property on="Save Michelson" class="Bool (strict)"("Visible"=w2453) -> ()  [unwired: 2 in, 2 out]
                                n1966 = property on="Acquire Michelson" class="Bool (strict)"("Visible"=TRUE) -> ()  [unwired: 2 in, 2 out]
                                n1967 = property on="Acquire Contrast" class="Bool (strict)"("Visible"=TRUE) -> ()  [unwired: 2 in, 2 out]
                                n1968 = property on="Save Contrast" class="Bool (strict)"("Visible"=w2453) -> ()  [unwired: 2 in, 2 out]
                                n1969 = property on="Pause Contrast" class="Bool (strict)"("Visible"=w2458) -> ()  [unwired: 2 in, 2 out]
                                n1970 = property on="Stop Contrast" class="Bool (strict)"("Visible"=w2458) -> ()  [unwired: 2 in, 2 out]
                                n1971 = property on="Elapsed (s)" class="DigNum (strict)"("Visible"=TRUE) -> ()  [unwired: 2 in, 2 out]
                                n1972 = property on="Michelson Expected (s)" class="DigNum (strict)"("Visible"=w2455) -> ()  [unwired: 2 in, 2 out]
                                n1973 = local read "Scan Contrast Ctrls"() -> (w2462:refnum<vi>[])
                                n1974 = control-ref of="MasterStop"() -> (w2451:refnum<vi>)
                                n1975 = control-ref of="MasterPause"() -> (w2452:refnum<vi>)
                                n1976 = property on="Michelson Elapsed (s)" class="DigNum (strict)"("Visible"=w2455) -> ()  [unwired: 2 in, 2 out]
                                n1977 = property on="Scan Michelson Progess Bar" class="Slide (strict)"("Visible"=w2455) -> ()  [unwired: 2 in, 2 out]
                                n1978 = control-ref of="ExperimentStopped?"() -> (w2450:refnum<vi>)
                                n1979 = call "CheckStopAndReset.vi"("ExperimentStopped?"=w2450, "MasterStop"=w2451, "MasterPause"=w2452) -> ()
                                n1980 = call "Enable&Disable_Controls.vi"("Enum"=enum16{"Enabled", "Disabled", "Disabled&Grayed"}."Enabled", "References"=w2462) -> ()  [unwired: 1 in]
                              }
                            }
                          }
                        }
                      }
                      frame "Acquire XY Map" {
                        n1981 = stacked-sequence {
                          frame #0 {
                            # "background"
                            n1982 = local read "Background taken?"() -> (w2466:bool)
                            n1983 = case shown="False" w2466 {
                              frame False {
                                n1984 = stacked-sequence {
                                tunnel: [_ _ w2516] -> w2467
                                frame #0 {
                                n1985 = local read "Log file"() -> (w2501:string)
                                n1986 = property on="CCD 1D Spectrum Main" class="XYGraph (strict)"("YScale.Offset"=0.0 ("Y Scale.Offset and Multiplier:Offset")) -> ()  [unwired: 2 in, 2 out]
                                n1987 = call "Write2LogFile.vi"("Add to log file"="Acquiring background", "Log file before"=w2501, "Checkbox"=FALSE) -> ("Log file after"=w2500:string)
                                n1988 = local write "Log file"(w2500) -> ()
                                }
                                frame #1 {
                                # "make sure shutter is closed"
                                n1989 = local read "KCube Shutter On?"() -> (w2502:bool)
                                n1990 = control-ref of="Shutter Ctrls"() -> (w2506:refnum<vi>)
                                n1991 = property class="Ring (strict)"(reference=w2506) -> ("Value"=w2505:u16)  [unwired: 1 in, 2 out]
                                n1992 = control-ref of="KCube Shutter Device Reference"() -> (w2507:refnum<vi>)
                                n1993 = Equal?(x=w2505, y=u16 0) -> (x = y?=w2503:bool)
                                n1994 = case shown="False" w2503 {
                                tunnel: w2507 -> [w2510 _]
                                tunnel: w2506 -> [w2509 _]
                                tunnel: w2502 -> [w2508 _]
                                frame False {
                                n1995 = call "Shutter.vi"("KCube Shutter Device Reference 2"=w2510, "Shutter Ctrls 2"=w2509, "Shutter on?"=w2508) -> ()
                                }
                                frame True {
                                }
                                }
                                }
                                frame #2 {
                                # "acquire"
                                n1996 = local read "LightField Automation error out"() -> (w2514:errorcluster)
                                n1997 = local read "LightField Automation out"() -> (w2515:refnum<class "LightField Automation.lvclass">)
                                n1998 = local read "Accumulations"() -> (w2511:dbl)
                                n1999 = call "LFA_Capture.vi"("error in (no error)"=w2514, "Frames"=w2511, "LightField Automation in"=w2515) -> ("error out"=w2513:errorcluster, "Data"=w2516:T26, "LightField Automation out"=w2512:refnum<class "LightField Automation.lvclass">)  [unwired: 6 in]
                                n2000 = local write "LightField Automation error out"(w2513) -> ()
                                n2001 = local write "LightField Automation out"(w2512) -> ()
                                }
                                }
                                n2002 = local read "Acq Mode"() -> (w2468:T3)
                                n2003 = case shown="\"Spectrum\", Default" w2468 {
                                selector: w2468 -> [w2469 w2487]
                                tunnel: w2467 -> [w2470 w2488]
                                frame "Spectrum", Default {
                                n2004 = stacked-sequence {
                                tunnel: w2470 -> [_ w2481 _ _]
                                tunnel: w2469 -> [_ w2479 _ _]
                                frame #0 {
                                n2005 = property on="CCD 2D Image Main" class="IntGraph (strict)"("Visible"=FALSE) -> ()  [unwired: 2 in, 2 out]
                                n2006 = property on="CCD 1D Spectrum Main" class="XYGraph (strict)"("Visible"=TRUE) -> ()  [unwired: 2 in, 2 out]
                                }
                                frame #1 {
                                n2007 = local read "Wavelength calibration"() -> (w2478:dbl[])
                                n2008 = local read "CCD ROI"() -> (w2474:T20)
                                n2009 = Divide(x=1239.842, y=w2478) -> (x/y=w2476:dbl[])
                                n2010 = call "PrepareData4Graph.vi"("Wavelength nm"=w2476, "DataLF"=w2481, "CCD ROI"=w2474, "AcqMode"=w2479, "Data type"=T30."Spectre") -> ("Spectrum"=w2480:cluster{"Array 2":dbl[], "Array":dbl[]}, "PLInt out"=w2473:dbl[])  [unwired: 2 in, 2 out]
                                n2011 = local write "CCD 1D Spectrum Main"(w2480) -> ()
                                n2012 = local write "BackgroundSpec"(w2473) -> ()